vi "UHR-Fleezers Control (host) - 12.4.vi"() -> ()   [LabVIEW 2012] (continued)
        n2469 = Build Array (concatenate)(w3745, w3711) -> (w3744:dbl[])
        n2470 = Select(t=w3713, s=w3710, f=w3772) -> (s? t:f=w3757:dbl[])
        n2471 = feedback-in #11(w3757) -> ()
        n2472 = Select(t=w3711, s=w3710, f=w3744) -> (s? t:f=w3729:dbl[])
        n2473 = feedback-in #12(w3729) -> ()
        n2474 = feedback #13(w3715) -> (w3866:dbl[])
        n2475 = Build Array (concatenate)(w3866, w3715) -> (w3848:dbl[])
        n2476 = Select(t=w3715, s=w3710, f=w3848) -> (s? t:f=w3852:dbl[])
        n2477 = feedback-in #13(w3852) -> ()
        n2478 = feedback #14(w3797) -> (w3854:dbl[])
        n2479 = Build Array (concatenate)(w3854, w3797) -> (w3845:dbl[])
        n2480 = feedback #15(w3804) -> (w3864:dbl[])
        n2481 = Build Array (concatenate)(w3864, w3804) -> (w3863:dbl[])
        n2482 = feedback #16(w3799) -> (w3856:dbl[])
        n2483 = Build Array (concatenate)(w3856, w3799) -> (w3857:dbl[])
        n2484 = Select(t=w3797, s=w3710, f=w3845) -> (s? t:f=w3801:dbl[])
        n2485 = feedback-in #14(w3801) -> ()
        n2486 = Select(t=w3804, s=w3710, f=w3863) -> (s? t:f=w3803:dbl[])
        n2487 = feedback-in #15(w3803) -> ()
        n2488 = Select(t=w3799, s=w3710, f=w3857) -> (s? t:f=w3802:dbl[])
        n2489 = feedback-in #16(w3802) -> ()
        n2490 = call "integrate 1D array interval - double.vi"("Ave N"=w3709, "Array In"=w3757) -> ("Array Out"=w3768:dbl[])  [unwired: 1 out]
        n2491 = call "integrate 1D array interval - double.vi"("Ave N"=w3709, "Array In"=w3729) -> ("Array Out"=w3740:dbl[])  [unwired: 1 out]
        n2492 = call "integrate 1D array interval - double.vi"("Ave N"=w3709, "Array In"=w3852) -> ("Array Out"=w3851:dbl[])  [unwired: 1 out]
        n2493 = Array Size(array=w3768) -> (size(s)=w3769:i32)
        n2494 = Array Size(array=w3740) -> (size(s)=w3741:i32)
        n2495 = Array Size(array=w3851) -> (size(s)=w3853:i32)
        n2496 = Multiply(x=w3707, y=w3708) -> (x*y=w3771:u64)
        n2497 = Multiply(x=w3707, y=w3708) -> (x*y=w3743:u64)
        n2498 = Multiply(x=w3707, y=w3708) -> (x*y=w3861:u64)
        n2499 = Subtract(x=w3771, y=w3769) -> (x-y=w3762:u64)
        n2500 = call-poly <vilib>:"Mean.vi"("X"=w3768) -> ("mean"=w3759:dbl)  [unwired: 1 out]
        n2501 = Subtract(x=w3743, y=w3741) -> (x-y=w3734:u64)
        n2502 = call-poly <vilib>:"Mean.vi"("X"=w3740) -> ("mean"=w3731:dbl)  [unwired: 1 out]
        n2503 = Subtract(x=w3861, y=w3853) -> (x-y=w3795:u64)
        n2504 = call-poly <vilib>:"Mean.vi"("X"=w3851) -> ("mean"=w3792:dbl)  [unwired: 1 out]
        n2505 = call-poly <vilib>:"Mean.vi"("X"=w3801) -> ("mean"=w3785:dbl)  [unwired: 1 out]
        n2506 = call-poly <vilib>:"Mean.vi"("X"=w3803) -> ("mean"=w3790:dbl)  [unwired: 1 out]
        n2507 = call-poly <vilib>:"Mean.vi"("X"=w3802) -> ("mean"=w3788:dbl)  [unwired: 1 out]
        n2508 = Initialize Array(1.0 ("element"), w3762) -> (w3758:dbl[])
        n2509 = Initialize Array(1.0 ("element"), w3734) -> (w3730:dbl[])
        n2510 = Initialize Array(1.0 ("element"), w3795) -> (w3786:dbl[])
        n2511 = Multiply(x=w3758, y=w3759) -> (x*y=w3760:dbl[])
        n2512 = Multiply(x=w3730, y=w3731) -> (x*y=w3732:dbl[])
        n2513 = Multiply(x=w3786, y=w3792) -> (x*y=w3793:dbl[])
        n2514 = Multiply(x=w3786, y=w3788) -> (x*y=w3789:dbl[])
        n2515 = Multiply(x=w3786, y=w3790) -> (x*y=w3791:dbl[])
        n2516 = Multiply(x=w3786, y=w3785) -> (x*y=w3787:dbl[])
        n2517 = Build Array (concatenate)(w3768, w3760) -> (w3770:dbl[])
        n2518 = Build Array (concatenate)(w3740, w3732) -> (w3742:dbl[])
        n2519 = Build Array (concatenate)(w3851, w3793) -> (w3860:dbl[])
        n2520 = Build Array (concatenate)(w3801, w3787) -> (w3855:dbl[])
        n2521 = Build Array (concatenate)(w3803, w3791) -> (w3859:dbl[])
        n2522 = Build Array (concatenate)(w3802, w3789) -> (w3858:dbl[])
        n2523 = Reshape Array(w3770, w3707, w3708) -> (w3766:dbl[][])
        n2524 = Reshape Array(w3742, w3707, w3708) -> (w3738:dbl[][])
        n2525 = Reshape Array(w3860, w3707, w3708) -> (w3838:dbl[][])
        n2526 = Reshape Array(w3855, w3707, w3708) -> (w3821:dbl[][])
        n2527 = Reshape Array(w3859, w3707, w3708) -> (w3813:dbl[][])
        n2528 = Reshape Array(w3858, w3707, w3708) -> (w3828:dbl[][])
        n2529 = Array Subset(array=w3766, index (col)=0 ("index"), length (col)=w3706) -> (w3765:dbl[][])  [unwired: 2 in]
        n2530 = Array Subset(array=w3766, index (col)=w3706) -> (w3763:dbl[][])  [unwired: 3 in]
        n2531 = Array Subset(array=w3738, index (col)=0 ("index"), length (col)=w3706) -> (w3737:dbl[][])  [unwired: 2 in]
        n2532 = Array Subset(array=w3738, index (col)=w3706) -> (w3735:dbl[][])  [unwired: 3 in]
        n2533 = Array Subset(array=w3828, index (col)=0 ("index"), length (col)=w3706) -> (w3833:dbl[][])  [unwired: 2 in]
        n2534 = Array Subset(array=w3828, index (col)=w3706) -> (w3831:dbl[][])  [unwired: 3 in]
        n2535 = Array Subset(array=w3838, index (col)=0 ("index"), length (col)=w3706) -> (w3837:dbl[][])  [unwired: 2 in]
        n2536 = Array Subset(array=w3838, index (col)=w3706) -> (w3835:dbl[][])  [unwired: 3 in]
        n2537 = Array Subset(array=w3813, index (col)=0 ("index"), length (col)=w3706) -> (w3819:dbl[][])  [unwired: 2 in]
        n2538 = Array Subset(array=w3813, index (col)=w3706) -> (w3817:dbl[][])  [unwired: 3 in]
        n2539 = Array Subset(array=w3821, index (col)=0 ("index"), length (col)=w3706) -> (w3826:dbl[][])  [unwired: 2 in]
        n2540 = Array Subset(array=w3821, index (col)=w3706) -> (w3824:dbl[][])  [unwired: 3 in]
        n2541 = for {
          tunnel: w3765 -> [w3870] mode=indexing
          tunnel: [w3869] -> w3764 mode=indexing
          workers-P: _ -> [_]
          n2542 = Reverse 1D Array(array=w3870) -> (reversed array=w3869:dbl[])
        }
        n2543 = for {
          tunnel: w3737 -> [w3868] mode=indexing
          tunnel: [w3867] -> w3736 mode=indexing
          workers-P: _ -> [_]
          n2544 = Reverse 1D Array(array=w3868) -> (reversed array=w3867:dbl[])
        }
        n2545 = for {
          tunnel: w3833 -> [w3876] mode=indexing
          tunnel: [w3875] -> w3832 mode=indexing
          workers-P: _ -> [_]
          n2546 = Reverse 1D Array(array=w3876) -> (reversed array=w3875:dbl[])
        }
        n2547 = for {
          tunnel: w3837 -> [w3878] mode=indexing
          tunnel: [w3877] -> w3836 mode=indexing
          workers-P: _ -> [_]
          n2548 = Reverse 1D Array(array=w3878) -> (reversed array=w3877:dbl[])
        }
        n2549 = for {
          tunnel: w3819 -> [w3872] mode=indexing
          tunnel: [w3871] -> w3818 mode=indexing
          workers-P: _ -> [_]
          n2550 = Reverse 1D Array(array=w3872) -> (reversed array=w3871:dbl[])
        }
        n2551 = for {
          tunnel: w3826 -> [w3874] mode=indexing
          tunnel: [w3873] -> w3825 mode=indexing
          workers-P: _ -> [_]
          n2552 = Reverse 1D Array(array=w3874) -> (reversed array=w3873:dbl[])
        }
        n2553 = Index Array(array=w3838, index (row)=0) -> (element=→"Waveform Graph":dbl[])  [unwired: 1 in]
        n2554 = Add(x=w3764, y=w3763) -> (x+y=w3750:dbl[][])
        n2555 = Add(x=w3736, y=w3735) -> (x+y=w3722:dbl[][])
        n2556 = Add(x=w3832, y=w3831) -> (x+y=w3830:dbl[][])
        n2557 = Add(x=w3836, y=w3835) -> (x+y=w3810:dbl[][])
        n2558 = Add(x=w3818, y=w3817) -> (x+y=w3816:dbl[][])
        n2559 = Add(x=w3825, y=w3824) -> (x+y=w3823:dbl[][])
        n2560 = Divide(x=w3816, y=2) -> (x/y=w3814:dbl[][])
        n2561 = Divide(x=w3830, y=2) -> (x/y=w3775:dbl[][])
        n2562 = To Single Precision Float(number=w3810) -> (single precision float=w3809:sgl[][])
        n2563 = To Single Precision Float(number=w3750) -> (single precision float=w3754:sgl[][])
        n2564 = To Single Precision Float(number=w3722) -> (single precision float=w3726:sgl[][])
        n2565 = Divide(x=w3823, y=2) -> (x/y=w3777:dbl[][])
        n2566 = Transpose 2D Array(2D array=w3814) -> (transposed array=→"Data map":dbl[][])
        n2567 = To Single Precision Float(number=w3775) -> (single precision float=w3781:sgl[][])
        n2568 = To Single Precision Float(number=w3777) -> (single precision float=w3778:sgl[][])
        n2569 = call "IMAQ ArrayToImage"("Image Pixels (Float)"=w3809, "Image"=w3747) -> ("Image Out"=w3812:T2)  [unwired: 8 in, 1 out]
        n2570 = call "IMAQ ArrayToImage"("Image Pixels (Float)"=w3754, "Image"=w3746) -> ("Image Out"=w3756:T2)  [unwired: 8 in, 1 out]
        n2571 = call "IMAQ ArrayToImage"("Image Pixels (Float)"=w3726, "Image"=w3718) -> ("Image Out"=w3728:T2)  [unwired: 8 in, 1 out]
        n2572 = call "IMAQ ArrayToImage"("Image Pixels (Float)"=w3781, "Image"=w3719) -> ("Image Out"=w3783:T2)  [unwired: 8 in, 1 out]
        n2573 = call "IMAQ Symmetry"("Type of Symmetry"=w3811, "Image Src"=w3812) -> ("Image Dst Out"=w3807:T2)  [unwired: 3 in, 1 out]
        n2574 = call "IMAQ ArrayToImage"("Image Pixels (Float)"=w3778, "Image"=w3720) -> ("Image Out"=w3780:T2)  [unwired: 8 in, 1 out]
        n2575 = call "IMAQ Symmetry"("Type of Symmetry"=w3755, "Image Src"=w3756) -> ("Image Dst Out"=w3752:T2)  [unwired: 3 in, 1 out]
        n2576 = call "IMAQ Symmetry"("Type of Symmetry"=w3727, "Image Src"=w3728) -> ("Image Dst Out"=w3724:T2)  [unwired: 3 in, 1 out]
        n2577 = call "IMAQ Symmetry"("Type of Symmetry"=w3782, "Image Src"=w3783) -> ("Image Dst Out"=→"Detection Laser X":T2)  [unwired: 3 in, 1 out]
        n2578 = call "IMAQ Symmetry"("Type of Symmetry"=w3779, "Image Src"=w3780) -> ("Image Dst Out"=→"Detection Laser Y":T2)  [unwired: 3 in, 1 out]
        n2579 = call "IMAQ Set Simple Calibration"("Calibration Axis Info"=T34 {"Origin Pixel"={"X"=0.0, "Y"=0.0}, "Angle Relative to Horizontal (deg)"=0.0, "Axis Reference"=0}, "Grid Descriptor"=T35 {"X Step"=0.3, "Y Step"=0.3, "Unit"=enum."Undefined"}, "Image"=w3807) -> ("Calibrated Image"=→"APD 1":T2)  [unwired: 7 in, 1 out]
        n2580 = call "IMAQ Set Simple Calibration"("Calibration Axis Info"=T34 {"Origin Pixel"={"X"=0.0, "Y"=0.0}, "Angle Relative to Horizontal (deg)"=0.0, "Axis Reference"=0}, "Grid Descriptor"=T35 {"X Step"=0.3, "Y Step"=0.3, "Unit"=enum."Undefined"}, "Image"=w3752) -> ("Calibrated Image"=→"APD 2":T2)  [unwired: 7 in, 1 out]
        n2581 = call "IMAQ Set Simple Calibration"("Calibration Axis Info"=T34 {"Origin Pixel"={"X"=0.0, "Y"=0.0}, "Angle Relative to Horizontal (deg)"=0.0, "Axis Reference"=0}, "Grid Descriptor"=T35 {"X Step"=0.3, "Y Step"=0.3, "Unit"=enum."Undefined"}, "Image"=w3724) -> ("Calibrated Image"=→"APD 3":T2)  [unwired: 7 in, 1 out]
      }
    }
    n2582 = case "For computing FFTs for display" shown="True" "Compute FFT" {
      tunnel: w3218 -> [_ w4350]
      frame False {
      }
      frame True {
        n2583 = Build Array("FFT 1 Choice 1", "FFT 1 Choice 2", "FFT 2 Choice 1", "FFT 2 Choice 2") -> (w4343:u16[])
        n2584 = Array Size(array=w4350) -> (size(s)=w4349:i32)
        n2585 = feedback-in #17(w4343) -> ()
        n2586 = feedback #17(u16[] [100, 100, 100, 100]) -> (w4344:u16[])
        n2587 = feedback-in #18("# Spectra to Ave.") -> ()
        n2588 = feedback #18("# Spectra to Ave.") -> (w4341:dbl)
        n2589 = Not Equal?(x="# Spectra to Ave.", y=w4341) -> (x != y?=w4340:bool)
        n2590 = Not Equal?(x=w4343, y=w4344) -> (x != y?=w4342:bool)
        n2591 = feedback #19(1.0) -> (w4327:dbl)
        n2592 = Compound Arithmetic op=OR("Reset FFT", w4342, w4340) -> (w4325:bool)
        n2593 = Select(t=1.0, s=w4325, f=w4327) -> (s? t:f=w4329:dbl)
        n2594 = Greater?(x=w4329, y="# Spectra to Ave.") -> (0:w4348:bool)
        n2595 = Increment(x=w4329) -> (x+1=w4328:dbl)
        n2596 = feedback-in #19(w4328) -> ()
        n2597 = local read "DMA Update Period (s)"() -> (w4323:dbl)
        n2598 = Multiply(x="# Spectra to Ave.", y=w4323) -> (x*y=→"Ave. Time (s)":dbl)
        n2599 = Build Array(cluster{"f0":dbl, "df":dbl, "magnitude":dbl[]} {"f0"=0.0, "df"=0.0, "magnitude"=[]} ("PSD")) -> (w4332:cluster{"f0":dbl, "df":dbl, "magnitude":dbl[]}[])
        n2600 = Build Array(w4332, w4332, w4332, w4332) -> (w4334:T44)
        n2601 = feedback #20(w4334) -> (w4339:T44)
        n2602 = for {
          N: 4 -> [_]
          tunnel: w4343 -> [w4372] mode=indexing
          tunnel: w4350 -> [w4373]
          tunnel: w4349 -> [w4375]
          tunnel: w4325 -> [w4368]
          tunnel: w4348 -> [w4367]
          tunnel: "# Spectra to Ave." -> [w4366]
          tunnel: [w4365] -> w4338 mode=indexing
          tunnel: w4339 -> [w4370] mode=indexing
          tunnel: [w4369] -> w4326 mode=indexing
          tunnel: w4329 -> [w4364]
          n2603 = Less?(x=w4372, y=w4375) -> (x < y?=w4374:bool)
          n2604 = Index Array(array=w4373, index=w4372) -> (element=w4371:waveform(dbl))
          n2605 = case shown="True" w4374 {
            tunnel: w4371 -> [_ w4392]
            tunnel: w4370 -> [w4377 w4390]
            tunnel: [w4377 w4378] -> w4369
            tunnel: w4368 -> [_ w4389]
            tunnel: w4367 -> [_ w4382]
            tunnel: w4366 -> [_ w4381]
            tunnel: [cluster{"f0":dbl, "df":dbl, "magnitude":dbl[]} {"f0"=0.0, "df"=0.0, "magnitude"=[]} ("PSD") w4383] -> w4365
            tunnel: w4364 -> [_ w4380]
            frame False {
            }
            frame True {
              n2606 = call <vilib>:"Std Deviation and Variance.vi"("X"=w4392) -> ("mean"=w4393:dbl)  [unwired: 1 in, 2 out]
              n2607 = Subtract(x=w4392, y=w4393) -> (x-y=w4391:waveform(dbl))
              n2608 = xnode "Spectral Measurements"("Signals"=w4391) -> ("PSD"=w4385:cluster{"f0":dbl, "df":dbl, "magnitude":dbl[]})  [unwired: 1 in, 1 out]
              n2609 = case shown="False" w4389 {
                tunnel: w4390 -> [w4402 _]
                tunnel: [w4398 w4407] -> w4378
                tunnel: w4385 -> [w4401 w4408]
                tunnel: w4382 -> [w4400 _]
                frame False {
                  n2610 = Build Array (concatenate)(w4402, w4401) -> (w4399:cluster{"f0":dbl, "df":dbl, "magnitude":dbl[]}[])
                  n2611 = case shown="True" w4400 {
                    tunnel: w4399 -> [w4403 w4406]
                    tunnel: [w4403 w4404] -> w4398
                    frame False {
                    }
                    frame True {
                      n2612 = Delete From Array(array=w4406, index=0) -> (array with subset deleted=w4404:cluster{"f0":dbl, "df":dbl, "magnitude":dbl[]}[])  [unwired: 1 in, 1 out]
                    }
                  }
                }
                frame True {
                  n2613 = Build Array(w4408) -> (w4407:cluster{"f0":dbl, "df":dbl, "magnitude":dbl[]}[])
                }
              }
              n2614 = for {
                tunnel: w4378 -> [w4397] mode=indexing
                tunnel: [w4396] -> w4388 mode=indexing
                workers-P: _ -> [_]
                n2615 = Unbundle By Name(w4397) -> ("magnitude"=w4396:dbl[])
              }
              n2616 = Transpose 2D Array(2D array=w4388) -> (transposed array=w4387:dbl[][])
              n2617 = for {
                tunnel: w4387 -> [w4395] mode=indexing
                tunnel: [w4394] -> w4386 mode=indexing
                workers-P: _ -> [_]
                n2618 = Add Array Elements(numeric array=w4395) -> (sum=w4394:dbl)
              }
              n2619 = Select(t=w4381, s=w4382, f=w4380) -> (s? t:f=w4379:dbl)
              n2620 = Divide(x=w4386, y=w4379) -> (x/y=w4384:dbl[])
              n2621 = Bundle By Name(cluster=w4385, "magnitude"=w4384) -> (w4383:cluster{"f0":dbl, "df":dbl, "magnitude":dbl[]})
            }
          }
        }
        n2622 = case shown="True" w4325 {
          tunnel: w4326 -> [w4357 w4363]
          tunnel: [w4357 w4358] -> w4324
          frame False {
          }
          frame True {
            n2623 = Array Subset(array=w4363, index (row)=0 ("index"), length (row)=4 ("length"), index (col)=0 ("index"), length (col)=1 ("length")) -> (w4358:T44)
          }
        }
        n2624 = feedback-in #20(w4324) -> ()
        n2625 = Split 1D Array(array=w4338, index=2) -> (first subarray=→"FFT 1":cluster{"f0":dbl, "df":dbl, "magnitude":dbl[]}[], second subarray=→"FFT 2":cluster{"f0":dbl, "df":dbl, "magnitude":dbl[]}[])
      }
    }
    n2626 = Index Array(array=w3216, index=4) -> (element=w3272:waveform(dbl))
    n2627 = Index Array(array=w3216, index=7) -> (element=w3269:waveform(dbl))
    n2628 = Divide(x="T1 offset_x (mV)", y=1000.0) -> (x/y=w3273:dbl)
    n2629 = feedback-in #21("Calibration") -> ()
    n2630 = feedback #21(u16 1 ("Calibration")) -> (w3291:u16)
    n2631 = Divide(x="T2 offset_x (mV)", y=1000.0) -> (x/y=w3271:dbl)
    n2632 = case shown="2" "Calibration" {
      tunnel: "T1 alpha_x (nm/V)" -> [_ w3671 w3692]
      tunnel: "T1 kappa_x (pN/nm)" -> [_ _ w3682]
      tunnel: "T2 alpha_x (nm/V)" -> [_ w3670 w3690]
      tunnel: "T2 kappa_x (pN/nm)" -> [_ _ w3683]
      tunnel: w3272 -> [w3653 w3668 w3688]
      tunnel: w3269 -> [w3652 w3666 w3686]
      tunnel: [w3653 w3665 w3685] -> w3300
      tunnel: [w3652 w3664 w3684] -> w3299
      tunnel: ["T1 X (V)" ("Label.Text") "T1 X (nm)" ("Label.Text") "T1 X (pN)" ("Label.Text")] -> w3288
      tunnel: ["T2 X (V)" ("Label.Text") "T2 X (nm)" ("Label.Text") "T2 X (pN)" ("Label.Text")] -> w3287
      tunnel: ["Position (V)" ("Label.Text") "Position (nm)" ("Label.Text") "Force (pN)" ("Label.Text")] -> w3289
      tunnel: w3271 -> [_ w3656 w3675]
      tunnel: w3273 -> [_ w3659 w3677]
      tunnel: ["Mean (V)" ("Label.Text") "Mean (nm)" ("Label.Text") "Mean (pN)" ("Label.Text")] -> w3284
      tunnel: ["Difference (V)" ("Label.Text") "Difference (nm)" ("Label.Text") "Difference (pN)" ("Label.Text")] -> w3224
      frame 0, Default {
      }
      frame 1 {
        n2633 = Unbundle By Name(w3668) -> ("Y"=w3672:dbl[])
        n2634 = Unbundle By Name(w3666) -> ("Y"=w3657:dbl[])
        n2635 = Subtract(x=w3672, y=w3659) -> (x-y=w3660:dbl[])
        n2636 = Subtract(x=w3657, y=w3656) -> (x-y=w3658:dbl[])
        n2637 = Multiply(x=w3658, y=w3670) -> (x*y=w3667:dbl[])
        n2638 = Multiply(x=w3671, y=w3660) -> (x*y=w3669:dbl[])
        n2639 = Bundle By Name(cluster=w3666, "Y"=w3667) -> (w3664:waveform(dbl))
        n2640 = Bundle By Name(cluster=w3668, "Y"=w3669) -> (w3665:waveform(dbl))
      }
      frame 2 {
        n2641 = Unbundle By Name(w3688) -> ("Y"=w3693:dbl[])
        n2642 = Unbundle By Name(w3686) -> ("Y"=w3691:dbl[])
        n2643 = Subtract(x=w3691, y=w3675) -> (x-y=w3676:dbl[])
        n2644 = Subtract(x=w3693, y=w3677) -> (x-y=w3678:dbl[])
        n2645 = Compound Arithmetic op=MULTIPLY(w3676, w3690, w3683) -> (w3687:dbl[])
        n2646 = Compound Arithmetic op=MULTIPLY(w3682, w3692, w3678) -> (w3689:dbl[])
        n2647 = Bundle By Name(cluster=w3686, "Y"=w3687) -> (w3684:waveform(dbl))
        n2648 = Bundle By Name(cluster=w3688, "Y"=w3689) -> (w3685:waveform(dbl))
      }
    }
    n2649 = case shown="True" "Read Lateness and Rel Phase" {
      tunnel: w3090 -> [w3602 w3641]
      tunnel: w3089 -> [w3603 w3640]
      tunnel: [w3602 w3607] -> w3266
      tunnel: [w3603 w3606] -> w3265
      frame False {
      }
      frame True {
        n2650 = xnode "Read/Write Control"("FPGA VI Reference In"=w3641, "error in"=w3640) -> ("FPGA VI Reference Out"=w3609:T19, "error out"=w3608:errorcluster, "GI Relative phase"=→"GI relative phase":i16, "Relative phase"=→"Relative phase (AI1)":i16, "AI Late Counter"=→"Late Counter (AI1)":u8, "GI Late Counter"=→"GI Late Counter":u8, "MCL Late Counter"=→"MCL Late Counter":u8, "MCL Relative Phase"=→"Relative Phase (MCL)":i16, "APD Acq Relative Phase"=→"APD Acq Relative Phase":i16, "APD 1 Gate Relative Phase"=→"APD 1 Gate Relative Phase":i16, "APD 2 Gate Relative Phase"=→"APD 2 Gate Relative Phase":i16, "APD Acq Late Counter"=→"APD Acq Late Counter":u8, "APD 1 Gate Late Counter"=→"APD 1 Gate Late Counter":u8, "APD 2 Gate Late Counter"=→"APD 2 Gate Late Counter":u8, "Green FB Relative Phase"=→"Relative phase (Green FB)":i16, "GI Relative phase 2"=→"GI relative phase 2":i16, "GI Late Counter 2"=→"GI Late Counter 2":u8, "Trap Pos FIFO Timeout"=→"Trap Pos FIFO Timeout":u16, "Trap AI FIFO Timeout"=→"Trap AI FIFO Timeout":u16, "RI Late Counter"=→"RI Late Counter":u8, "RI Late Counter 2"=→"RI Late Counter 2":u8, "RI Relative phase"=→"RI relative phase":i16, "RI Relative phase 2"=→"RI relative phase 2":i16, "Red FB Relative Phase"=→"Relative phase (RI FB)":i16, "Red Late Counter"=→"Red AI Late Counter":u8, "Green Late Counter"=→"Green AI Late Counter":u8, "BI Late Counter (AO)"=→"Late Counter (BI AO)":u8, "Blue Late Counter (D)"=→"Late Counter (BI DO)":u8, "Blue Int Late Counter"=→"Late Counter (BI AI)":u8, "Blue Int Relative Phase"=→"Relative phase (BI AI)":i16, "BI Relative phase (AO)"=→"Relative phase (BI AO)":i16, "BI Relative phase (D)"=→"Relative phase (BI DO)":i16)
        n2651 = xnode "Read/Write Control"("FPGA VI Reference In"=w3609, "error in"=w3608) -> ("FPGA VI Reference Out"=w3607:T19, "error out"=w3606:errorcluster, "APD 3 Gate Late Counter"=→"APD 3 Gate Late Counter":u8, "APD 3 Gate Relative Phase"=→"APD 3 Gate Relative Phase":i16)
      }
    }
    n2652 = Not Equal?(x=w3291, y="Calibration") -> (x != y?=w3250:bool)
    n2653 = case shown="True" w3250 {
      tunnel: w3289 -> [_ w3646]
      tunnel: w3288 -> [_ w3645]
      tunnel: w3287 -> [_ w3644]
      tunnel: w3284 -> [_ w3643]
      tunnel: w3224 -> [_ w3642]
      frame False {
      }
      frame True {
        n2654 = property on="Force" class="WFChart (strict)"("YScale.NameLbl.Text"=w3646) -> ()  [unwired: 2 in, 2 out]
        n2655 = property on="T2 X" class="DigNum (strict)"("Caption.Text"=w3644) -> ()  [unwired: 2 in, 2 out]
        n2656 = property on="T1 X" class="DigNum (strict)"("Caption.Text"=w3645) -> ()  [unwired: 2 in, 2 out]
        n2657 = property on="Mean" class="DigNum (strict)"("Caption.Text"=w3643) -> ()  [unwired: 2 in, 2 out]
        n2658 = property on="Difference" class="DigNum (strict)"("Caption.Text"=w3642) -> ()  [unwired: 2 in, 2 out]
      }
    }
    n2659 = Unbundle By Name(w3272) -> ("Y"=w3275:dbl[])
    n2660 = Unbundle By Name(w3269) -> ("Y"=w3278:dbl[])
    n2661 = Subtract(x=w3275, y=w3273) -> (x-y=w3276:dbl[])
    n2662 = Subtract(x=w3278, y=w3271) -> (x-y=w3277:dbl[])
    n2663 = Multiply(x=w3277, y="T2 alpha_x (nm/V)") -> (x*y=w3072:dbl[])
    n2664 = Multiply(x="T1 alpha_x (nm/V)", y=w3276) -> (x*y=w3073:dbl[])
    n2665 = Not(x="Trap Trig. Fl.") -> (.not. x?=w3109:bool)
    n2666 = Multiply(x=w3299, y=-1.0) -> (x*y=w3280:waveform(dbl))
    n2667 = Subtract(x=w3073, y=w3072) -> (x-y=w3268:dbl[])
    n2668 = Unbundle By Name(w3299) -> ("Y"=w3240:dbl[])
    n2669 = Unbundle By Name(w3300) -> ("Y"=w3074:dbl[])
    n2670 = Negate(x=w3268) -> (-x=w3070:dbl[])
    n2671 = Build Array(w3300, w3280) -> (→"Force":waveform(dbl)[])
    n2672 = Subtract(x=w3070, y="Offset (nm)") -> (x-y=w3238:dbl[])
    n2673 = call-poly <vilib>:"Mean.vi"("X"=w3240) -> ("mean"=w3076:dbl)  [unwired: 1 out]
    "T2 X" <- w3076
    n2674 = Negate(x=w3240) -> (-x=w3241:dbl[])
    n2675 = call-poly <vilib>:"Mean.vi"("X"=w3074) -> ("mean"=w3077:dbl)  [unwired: 1 out]
    "T1 X" <- w3077
    n2676 = Negate(x=w3076) -> (-x=w3075:dbl)
    n2677 = Bundle By Name(cluster=w3272, "Y"=w3238) -> (w3215:waveform(dbl))
    "Bead Separation" <- w3215
    n2678 = Add(x=w3074, y=w3241) -> (x+y=w3242:dbl[])
    n2679 = Add(x=w3077, y=w3075) -> (x+y=w3286:dbl)
    n2680 = Subtract(x=w3077, y=w3075) -> (x-y=→"Difference":dbl)
    n2681 = Divide(x=w3242, y=2.0) -> (x/y=→"Vec Mean of T1 T2":dbl[])
    n2682 = Divide(x=w3286, y=2.0) -> (x/y=w3244:dbl)
    "Mean" <- w3244
    n2683 = feedback-in #22("Trap Trig. Fl.") -> ()
    n2684 = feedback #22("Trap Trig. Fl.") -> (w3107:bool)
    n2685 = And(x=w3109, y=w3107) -> (x .and. y?=w3108:bool)
    n2686 = case "If have just turned off triggering" shown="True" w3108 {
      tunnel: w3090 -> [_ w3437]
      tunnel: w3089 -> [_ w3436]
      frame False {
      }
      frame True {
        w3435 = FALSE ("FPGA Trap Trig")
        n2687 = xnode "Read/Write Control"("FPGA VI Reference In"=w3437, "error in"=w3436, "FPGA Trap Trig"=w3435) -> ("FPGA VI Reference Out"=w3434:T19, "error out"=w3433:errorcluster)
        n2688 = xnode "Read/Write Control"("FPGA VI Reference In"=w3434, "error in"=w3433, "TTrig?"=w3435) -> ()  [unwired: 2 out]
        n2689 = local write "Initializing"(FALSE ("Initializing")) -> ()
        n2690 = local write "Triggered"(FALSE ("Triggered")) -> ()
        n2691 = local write "Waiting"(FALSE ("Waiting")) -> ()
      }
    }
    n2692 = Not(x=w3107) -> (.not. x?=w3120:bool)
    n2693 = And(x="Trap Trig. Fl.", y=w3120) -> (x .and. y?=w3117:bool)
    n2694 = local read "Tether"() -> (w3245:bool)
    n2695 = Or(x=w3117, y="Reinitialize") -> (x .or. y?=w3103:bool)
    n2696 = feedback #23(w3113) -> (w3118:string)
    n2697 = Select(t=w3113, s=w3117, f=w3118) -> (s? t:f=w3112:string)
    n2698 = Select(t=w3113, s="Reinitialize", f=w3112) -> (s? t:f=w3111:string)
    n2699 = feedback #24(0) -> (w3115:i32)
    n2700 = feedback #25(w3238) -> (w3237:dbl[])
    n2701 = Build Array (concatenate)(w3238, w3237) -> (w3071:dbl[])
    n2702 = case "For determining if there is a tether still" shown="True" w3245 {
      tunnel: w3244 -> [_ w3561]
      frame False {
      }
      frame True {
        n2703 = Greater?(x="Lost Tether Alarm Threshold (pN)", y=w3561) -> (0:w3559:bool)
        n2704 = case shown="True" w3559 {
          frame False {
          }
          frame True {
            w3562 = FALSE ("Value (Signaling)")
            n2705 = flat-sequence {
              frame #0 {
                # "stop only if saving"
                n2706 = local read "Saving..."() -> (w3574:bool)
                n2707 = And(x=w3574, y="TA Cancel Save?") -> (x .and. y?=w3573:bool)
                n2708 = local write "Stop Saving"(w3573) -> ()
              }
              frame #1 {
                n2709 = case shown="True" "TA Green Off?" {
                  frame False {
                  }
                  frame True {
                    w3577 = FALSE ("Fl. Triggered...")
                    n2710 = local write "Fl. Triggered..."(w3577) -> ()
                    n2711 = property on="Green Laser ON" class="Bool (strict)"("Val(Sgnl)"=w3577) -> ()  [unwired: 2 in, 2 out]
                  }
                }
              }
            }
            n2712 = local read "Time tether formed"() -> (w3568:timestamp)
            n2713 = Get Date/Time In Seconds() -> (seconds since 1Jan1904=w3569:timestamp)
            n2714 = Subtract(x=w3569, y=w3568) -> (x-y=w3567:dbl)
            n2715 = Number To Decimal String(number=w3567) -> (decimal integer string=w3564:string)  [unwired: 1 out]
            n2716 = local read "Messages"() -> (w3571:string)
            n2717 = call <vilib>:"Beep.vi"() -> ()  [unwired: 3 in, 9 out]
            n2718 = Concatenate Strings("Lost tether (" ("Message to add"), w3564, " s)." ("string")) -> (w3566:string)
            n2719 = local write "Tether"(FALSE ("Tether")) -> ()
            n2720 = call "Update messages.vi"("Message to add"=w3566, "Old message string"=w3571) -> ("New message string"=w3570:string)
            n2721 = local write "Messages"(w3570) -> ()
            n2722 = property on="Fl. Triggered..." class="Bool (strict)"("Val(Sgnl)"=w3562) -> ()  [unwired: 2 in, 2 out]
            n2723 = local write "Dip for Protein"(w3562) -> ()
            n2724 = property on="Trap Pos. FB ON" class="Bool (strict)"("Val(Sgnl)"=w3562) -> ()  [unwired: 2 in, 2 out]
            n2725 = property on="Trap Trig. Fl." class="Bool (strict)"("Val(Sgnl)"=w3562) -> ()  [unwired: 2 in, 2 out]
          }
        }
      }
    }
    n2726 = case "For triggering actions based on the trap position (e.g., turning the excitation laser on if trap under feedback moves so far)" shown="True" "Trap Trig. Fl." {
      tunnel: w3098 -> [_ w3450]
      tunnel: w3111 -> [_ w3449]
      tunnel: ["" ("t") w3448] -> w3119
      tunnel: w3103 -> [_ w3447]
      tunnel: [0 ("t") w3446] -> w3116
      tunnel: w3115 -> [_ w3445]
      tunnel: w3090 -> [_ w3444]
      tunnel: w3089 -> [_ w3443]
      frame False {
      }
      frame True {
        n2727 = case shown="\"Wait for trigger\"" w3449 {
          tunnel: w3450 -> [w3467 _ _ w3515]
          tunnel: [w3464 w3496 "" ("t") w3518] -> w3448
          tunnel: w3447 -> [_ _ _ w3506]
          tunnel: [w3463 w3493 0 ("t") w3507] -> w3446
          tunnel: w3445 -> [_ w3495 _ w3513]
          tunnel: w3444 -> [w3452 w3490 _ w3509]
          tunnel: w3443 -> [w3451 w3489 _ w3508]
          frame "Wait for trigger" {
            n2728 = local read "Trap Trig. (FPGA)"() -> (w3455:bool)
            n2729 = Subtract(x=w3467, y="Mean T1 Position\nto compare (nm)") -> (x-y=w3460:dbl[])
            n2730 = call <vilib>:"Std Deviation and Variance.vi"("X"=w3460) -> ("mean"=→"mean":dbl, "standard deviation"=→"standard\ndeviation":dbl)  [unwired: 1 in, 1 out]
            n2731 = Array Max & Min(array=w3460) -> (max value=→"max value":dbl, min value=→"min value":dbl)  [unwired: 2 out]
            n2732 = Greater?(x=w3460, y="Threshold (nm)") -> (0:w3470:bool[])
            n2733 = case shown="True" w3455 {
              tunnel: w3452 -> [_ w3476]
              tunnel: w3451 -> [_ w3475]
              tunnel: [FALSE ("TTrig?") w3474] -> w3458
              frame False {
              }
              frame True {
                n2734 = xnode "Read/Write Control"("FPGA VI Reference In"=w3476, "error in"=w3475) -> ("TTrig?"=w3474:bool)  [unwired: 2 out]
              }
            }
            n2735 = Or Array Elements(Boolean array=w3470) -> (logical OR=w3457:bool)
            n2736 = Select(t=w3458, s=w3455, f=w3457) -> (s? t:f=w3456:bool)
            n2737 = Not(x=w3455) -> (.not. x?=w3454:bool)
            n2738 = And(x=w3456, y=w3454) -> (x .and. y?=w3453:bool)
            n2739 = Select(t="Triggered", s=w3456, f="Wait for trigger") -> (s? t:f=w3464:string)
            n2740 = case shown="True" w3456 {
              tunnel: [0 0] -> w3463
              tunnel: w3452 -> [_ w3481]
              tunnel: w3451 -> [_ w3480]
              frame False {
                "Waiting" <- TRUE ("Waiting")
              }
              frame True {
                n2741 = xnode "Read/Write Control"("FPGA VI Reference In"=w3481, "error in"=w3480, "TTrig?"=FALSE) -> ()  [unwired: 2 out]
                n2742 = local read "Messages"() -> (w3484:string)
                n2743 = call <vilib>:"Beep.vi"() -> ()  [unwired: 12 in]
                n2744 = call "Update messages.vi"("Message to add"="Unwinding trigger.", "Old message string"=w3484) -> ("New message string"=w3485:string)
                n2745 = local write "Messages"(w3485) -> ()
                n2746 = local write "Waiting"(FALSE ("Waiting")) -> ()
                "Triggered" <- TRUE ("Triggered")
              }
            }
            n2747 = case "Only need to turn on laser if host triggered" shown="True" w3453 {
              frame False {
              }
              frame True {
                n2748 = property on="Green Laser ON" class="Bool (strict)"("Val(Sgnl)"=TRUE ("Value (Signaling)")) -> ()  [unwired: 2 in, 2 out]
              }
            }
          }
          frame "Triggered" {
            n2749 = local read "Trap Trig. (FPGA)"() -> (w3492:bool)
            n2750 = Increment(x=w3495) -> (x+1=w3493:i32)
            n2751 = Greater Or Equal?(x=w3493, y="Fl. ON time (n)") -> (x >= y?=w3491:bool)
            n2752 = Select(t="Wait for trigger", s=w3491, f="Triggered" ("t")) -> (s? t:f=w3496:string)
            n2753 = And(x=w3491, y=w3492) -> (x .and. y?=w3488:bool)
            n2754 = case shown="True" w3488 {
              tunnel: w3490 -> [_ w3500]
              tunnel: w3489 -> [_ w3499]
              frame False {
              }
              frame True {
                n2755 = xnode "Read/Write Control"("FPGA VI Reference In"=w3500, "error in"=w3499, "FPGA Trap Trig"=TRUE) -> ()  [unwired: 2 out]
              }
            }
            n2756 = case shown="True" w3491 {
              frame False {
              }
              frame True {
                w3502 = FALSE ("Value (Signaling)")
                n2757 = local write "Triggered"(w3502) -> ()
                n2758 = local write "Waiting"(TRUE ("Waiting")) -> ()
                n2759 = property on="Green Laser ON" class="Bool (strict)"("Val(Sgnl)"=w3502) -> ()  [unwired: 2 in, 2 out]
              }
            }
          }
          frame "Do nothing" {
          }
          frame "Initialize", Default {
            n2760 = Increment(x=w3513) -> (x+1=w3517:i32)
            n2761 = Select(t=1, s=w3506, f=w3517) -> (s? t:f=w3507:i32)
            n2762 = feedback #26(w3515) -> (w3521:dbl[])
            n2763 = Build Array (concatenate)(w3515, w3521) -> (w3514:dbl[])
            n2764 = Greater Or Equal?(x=w3507, y="Wait to get offset (n)") -> (x >= y?=w3510:bool)
            n2765 = Select(t=w3515, s=w3506, f=w3514) -> (s? t:f=w3516:dbl[])
            n2766 = feedback-in #26(w3516) -> ()
            n2767 = call-poly <vilib>:"Mean.vi"("X"=w3516) -> ("mean"=w3511:dbl)  [unwired: 1 out]
            n2768 = local write "Mean T1 Position\nto compare (nm)"(w3511) -> ()
            n2769 = case shown="True" w3506 {
              tunnel: w3509 -> [_ w3527]
              tunnel: w3508 -> [_ w3526]
              frame False {
              }
              frame True {
                w3523 = FALSE ("FPGA Trap Trig")
                n2770 = xnode "Read/Write Control"("FPGA VI Reference In"=w3527, "error in"=w3526, "FPGA Trap Trig"=w3523) -> ("FPGA VI Reference Out"=w3525:T19, "error out"=w3524:errorcluster)
                n2771 = xnode "Read/Write Control"("FPGA VI Reference In"=w3525, "error in"=w3524, "TTrig?"=w3523) -> ()  [unwired: 2 out]
              }
            }
            n2772 = Select(t="Wait for trigger", s=w3510, f="Initialize") -> (s? t:f=w3518:string)
            n2773 = case shown="True" w3510 {
              tunnel: w3511 -> [_ w3530]
              tunnel: w3509 -> [_ w3539]
              tunnel: w3508 -> [_ w3538]
              frame False {
                n2774 = local write "Waiting"(FALSE ("Waiting")) -> ()
                "Initializing" <- TRUE ("Initializing")
              }
              frame True {
                n2775 = local read "Threshold (nm)"() -> (w3542:dbl)
                n2776 = local read "AOM X Cal (nm/MHz)"() -> (w3541:dbl)
                n2777 = Add(x=w3530, y=w3542) -> (x+y=w3543:dbl)
                n2778 = Divide(x=w3543, y=w3541) -> (x/y=w3540:dbl)
                n2779 = call "IR AOM freq to word.vi"("Frequency In (MHz)"=w3540) -> ("Frequency Word Out (double)"=w3537:dbl)
                n2780 = local write "Initializing"(FALSE ("Initializing")) -> ()
                n2781 = local write "Waiting"(TRUE ("Waiting")) -> ()
                n2782 = To Quad Integer(1:w3537) -> (0:w3536:i64)
                n2783 = xnode "Read/Write Control"("FPGA VI Reference In"=w3539, "error in"=w3538, "FPGA TTrig Thresh"=w3536) -> ("FPGA VI Reference Out"=w3533:T19, "error out"=w3532:errorcluster)
                n2784 = xnode "Read/Write Control"("FPGA VI Reference In"=w3533, "error in"=w3532, "FPGA Trap Trig"=TRUE) -> ()  [unwired: 2 out]
              }
            }
          }
        }
      }
    }
    n2785 = feedback-in #23(w3119) -> ()
    n2786 = feedback-in #24(w3116) -> ()
    n2787 = Split 1D Array(array=w3071, index=w3133) -> (first subarray=w3234:dbl[])  [unwired: 1 out]
    n2788 = feedback-in #25(w3234) -> ()
    n2789 = call-poly <vilib>:"Mean.vi"("X"=w3234) -> ("mean"=w3233:dbl)  [unwired: 1 out]
    "Bead Mean (nm)" <- w3233
    n2790 = Subtract(x=w3234, y=w3233) -> (x-y=w3232:dbl[])
    n2791 = Square(x=w3232) -> (x^2=w3231:dbl[])
    n2792 = call-poly <vilib>:"Mean.vi"("X"=w3231) -> ("mean"=w3230:dbl)  [unwired: 1 out]
    n2793 = Square Root(x=w3230) -> (sqrt(x)=w3229:dbl)
    n2794 = Multiply(x=10.0, y=w3229) -> (x*y=→"RMS (Ang)":dbl)
    n2795 = xnode ("Read/Write Control")("FPGA VI Reference In"=w3266, "error in"=w3265) -> ("FPGA VI Reference Out"=w3101:T19, "error out"=w3100:errorcluster, "AI2 Y Sum Set 1"=w3364:i16, "AI2 Y Sum Set 2"=w3363:i16, "AI1 X Set 1"=w3165:fxp<+/-,16,1>, "AI1 X Set 2"=w3164:fxp<+/-,16,1>, "Trap Pos FB Int Signal"=→"Trap Pos FB Int Signal":fxp<+/-,24,9>, "Trap Pos FB Int-Norm Signal"=→"Trap Pos FB Int-Norm Signal":fxp<+/-,16,1>, "Trap Pos FB Action"=w3158:i64, "Scanning"=→"AOD Scanning":bool, "Scan I"=→"AOD Scan I":u64, "Scanning MCL"=w3366:bool, "Scan I (MCL)"=→"MCL Scan I":u64, "Green FB Sum"=w3303:i16, "Trap Pos FB Action"=w3088:i64, "TTrig Fin Thresh"=w3084:i64, "Red FB Intensity"=w3065:i16, "Blue Intensity"=w3060:i16)
    "MCL Scanning" <- w3366
    "Trap Pos FB Action" <- w3158
    n2796 = Divide(x=w3065, y=3276.7) -> (x/y=w3064:dbl)
    "Red laser intensity (V)" <- w3064
    n2797 = Divide(x=w3060, y=3276.7) -> (x/y=w3059:dbl)
    "Blue laser intensity (V)" <- w3059
    n2798 = Divide(x=w3303, y=3276.7) -> (x/y=w3063:dbl)
    "Green laser intensity (V)" <- w3063
    n2799 = local read "FB Trig Integrate"() -> (w3082:u32)
    n2800 = Divide(x=w3088, y=w3082) -> (x/y=w3081:dbl)
    "TTrig Sig (Int)" <- w3081
    n2801 = Bundle(w3063, w3064, w3059) -> (→"Fluorescence laser intensities plot":cluster{dbl, dbl, dbl})  [unwired: 1 in]
    n2802 = Divide(x=w3084, y=w3082) -> (x/y=w3079:dbl)
    "TTrig Fin Thresh (Int)" <- w3079
    n2803 = local read "AOM X Cal (nm/MHz)"() -> (w3087:dbl)
    n2804 = local read "AI2 (V)"() -> (w3365:cluster{"Set 1":dbl, "Set 2":dbl})
    n2805 = Bundle By Name(cluster=w3365, "Set 1"=w3364, "Set 2"=w3363) -> (w3361:cluster{"Set 1":dbl, "Set 2":dbl})
    n2806 = Divide(x=w3158, y=327.67) -> (x/y=→"Action (%)":dbl)
    n2807 = local read "Trap X (AI1)"() -> (w3178:T10)
    n2808 = call "IR AOM word double to freq.vi"("Frequency Word In (double)"=w3079) -> ("Frequency Out (MHz)"=w3078:dbl)
    n2809 = call "IR AOM word double to freq.vi"("Frequency Word In (double)"=w3081) -> ("Frequency Out (MHz)"=w3080:dbl)
    n2810 = Divide(x=w3361, y=3276.7) -> (x/y=w3360:cluster{"Set 1":dbl, "Set 2":dbl})
    n2811 = Multiply(x=w3080, y=w3087) -> (x*y=w3086:dbl)
    "TTrig Sig (nm)" <- w3086
    n2812 = Multiply(x=w3078, y=w3087) -> (x*y=w3085:dbl)
    "TTrig Fin Thresh (nm)" <- w3085
    n2813 = local write "AI2 (V)"(w3360) -> ()
    n2814 = Bundle(cluster=w3178, "Trap 1"=w3165, "Trap 2"=w3164) -> (→"Trap X (AI1)":T10)
    n2815 = Bundle(w3086, w3085) -> (→"TTrig":cluster{dbl, dbl})  [unwired: 1 in]
    n2816 = flat-sequence "To save data" {
      tunnel: [w4456] -> w3384
      tunnel: [w4457] -> w3383
      tunnel: w3334 -> [w4450]
      tunnel: w3106 -> [w4454]
      tunnel: ["Save Calibration"] -> w3357
      tunnel: w3354 -> [w4453]
      tunnel: [w4446] -> w3353
      tunnel: [w4443] -> w3352
      tunnel: [w4440] -> w3351
      tunnel: w3333 -> [w4442]
      tunnel: w3248 -> [w4436]
      tunnel: [w4436] -> w3247
      tunnel: ["Start Saving"] -> w3217
      tunnel: [w4430] -> w3146
      tunnel: [w4429] -> w3145
      tunnel: w3384 -> [w4693]
      tunnel: w3383 -> [w4692]
      tunnel: w3147 -> [w4691]
      tunnel: w3357 -> [w4690]
      tunnel: w3353 -> [w4688]
      tunnel: w3352 -> [w4687]
      tunnel: w3351 -> [w4686]
      tunnel: w3226 -> [w4685]
      tunnel: w3258 -> [w4684]
      tunnel: w3247 -> [w4683]
      tunnel: w3217 -> [w4682]
      tunnel: w3215 -> [w4681]
      tunnel: w3043 -> [w4680]
      tunnel: w3146 -> [w4679]
      tunnel: w3145 -> [w4678]
      tunnel: w3144 -> [w4677]
      tunnel: w3067 -> [w4676]
      frame #0 {
        n2817 = Or(x="Save N Sets", y="Start Saving") -> (x .or. y?=w4437:bool)
        n2818 = To Double Precision Float(number=w4453) -> (double precision float=w4447:dbl)
        n2819 = Build Array(w4437, "Save Calibration", w4450, w4442) -> (w4452:bool[])
        n2820 = Compound Arithmetic op=OR("Save Calibration", w4450, w4437, w4442) -> (w4455:bool)
        n2821 = Boolean Array To Number(Boolean array=w4452) -> (number=w4449:u32)
        n2822 = feedback #27(FALSE ("Save APD Data\nwith Trap Data")) -> (w4431:bool)
        n2823 = feedback #28(refnum<k0> refnum) -> (w4458:refnum<file>)
        n2824 = feedback #29(refnum<k0> refnum) -> (w4433:refnum<file>)
        n2825 = feedback #30(FALSE ("Save APD Data\nwith Trap Data")) -> (w4441:bool)
        n2826 = feedback #31(refnum<k0> refnum) -> (w4444:refnum<file>)
        n2827 = feedback #32(0) -> (w4460:i32)
        n2828 = feedback #33() -> (w4448:u32)  [unwired: 1 out]
        n2829 = case shown="True" w4455 {
          tunnel: [w4467 1] -> w4456
          tunnel: w4460 -> [w4469 _]
          tunnel: [w4468 w4487] -> w4457
          tunnel: w4458 -> [w4468 _]
          tunnel: w4454 -> [_ w4507]
          tunnel: w4447 -> [_ w4505]
          tunnel: w4449 -> [_ w4508]
          tunnel: [w4466 w4486] -> w4446
          tunnel: w4448 -> [w4466 _]
          tunnel: [w4465 w4484] -> w4443
          tunnel: w4444 -> [w4465 _]
          tunnel: [w4464 w4483] -> w4440
          tunnel: w4441 -> [w4464 _]
          tunnel: "Start Saving" -> [_ w4481]
          tunnel: w4436 -> [_ w4480]
          tunnel: [w4463 w4471] -> w4429
          tunnel: w4433 -> [w4463 _]
          tunnel: [w4462 w4470] -> w4430
          tunnel: w4431 -> [w4462 _]
          frame False {
            n2830 = Increment(x=w4469) -> (x+1=w4467:i32)
          }
          frame True {
            w4477 = FALSE ("Start Saving")
            w4482 = 9.0  # File Version
            w4490 = FALSE ("prepend array or string size? (T)")
            w4488 = T26."big-endian, network order" ("byte order (0:big-endian, network order)")
            n2831 = local read "BD 1 Frequency 1 (MHz)"() -> (w4504:dbl)
            n2832 = local read "BD 2 Frequency 1 (MHz)"() -> (w4503:dbl)
            n2833 = local read "BD 1 Frequency 2 (MHz)"() -> (w4502:dbl)
            n2834 = local read "BD 2 Frequency 2 (MHz)"() -> (w4501:dbl)
            n2835 = local read "BD 1 Frequency 3 (MHz)"() -> (w4500:dbl)
            n2836 = local read "BD 2 Frequency 3 (MHz)"() -> (w4499:dbl)
            n2837 = Array Size(array=w4480) -> (size(s)=w4479:i32)
            n2838 = To Double Precision Float(number=w4479) -> (double precision float=w4478:dbl)
            n2839 = local write "Save Calibration"(w4477) -> ()
            n2840 = local write "Start Saving"(w4477) -> ()
            n2841 = Build Array("Save APD Data\nwith Trap Data", "Save Trap Pos. Data") -> (w4474:bool[])
            n2842 = Boolean Array To Number(Boolean array=w4474) -> (number=w4473:u32)
            n2843 = Build Array(w4504, w4503, w4502, w4501, w4500, w4499) -> (w4498:dbl[])
            n2844 = case shown="1, Default" w4508 {
              tunnel: w4507 -> [w4580 w4600 w4616 w4654]
              tunnel: w4478 -> [w4585 w4607 w4636 w4673]
              tunnel: w4505 -> [w4584 w4606 w4635 w4672]
              tunnel: [w4581 w4602 w4627 w4664] -> w4496
              tunnel: [w4572 "Cal sets to save" w4617 w4655] -> w4486
              tunnel: w4498 -> [w4582 w4603 w4629 w4666]
              tunnel: "Save APD Data\nwith Trap Data" -> [w4579 _ w4613 w4652]
              tunnel: [w4579 w4594 w4613 w4652] -> w4483
              tunnel: w4482 -> [w4575 w4595 w4611 w4650]
              tunnel: w4481 -> [w4574 _ _ _]
              tunnel: [w4565 w4594 w4610 w4640] -> w4470
              tunnel: "Save Trap Pos. Data" -> [w4565 _ w4610 w4640]
              tunnel: w4473 -> [w4564 _ w4609 w4639]
              frame 1, Default {
                # "timeseries"
                n2845 = case shown="True" "Profile" {
                  tunnel: [w4588 w4592] -> w4569
                  tunnel: [w4588 w4591] -> w4568
                  tunnel: [w4588 w4590] -> w4567
                  tunnel: [w4588 w4589] -> w4566
                  frame False {
                    w4588 = 0.0 ("f")
                  }
                  frame True {
                    n2846 = local read "Current Position"() -> (w4593:cluster{dbl, dbl, dbl})
                    n2847 = local read "Y change (mm)"() -> (w4589:dbl)
                    n2848 = Unbundle(w4593) -> (w4592:dbl, w4591:dbl, w4590:dbl)
                  }
                }
                n2849 = local read "Save ave N"() -> (w4587:dbl)
                n2850 = Multiply(x=w4587, y=w4580) -> (x*y=w4586:dbl)
                n2851 = To Double Precision Float(number=w4564) -> (double precision float=w4578:dbl)
                n2852 = Build Array(w4575, w4580, w4586, w4585, w4584, 0.0 ("f")) -> (w4583:dbl[])
                n2853 = Build Array(w4578, w4569, w4568, w4567, w4566) -> (w4576:dbl[])
                n2854 = Select(t=u32 4000000000, s=w4574, f="N sets to save") -> (s? t:f=w4572:u32)
                n2855 = Build Array (concatenate)(w4583, w4582, w4576) -> (w4581:dbl[])
              }
              frame 2 {
                w4597 = 0.0 ("f")
                w4594 = FALSE ("Save APD Data\nwith Trap Data")
                # "calibration"
                n2856 = Boolean To (0,1)(Boolean=w4594) -> (0, 1=w4599:i16)
                n2857 = To Double Precision Float(number=w4599) -> (double precision float=w4598:dbl)
                n2858 = Build Array(w4598, w4597, w4597, w4597, w4597) -> (w4596:dbl[])
                n2859 = Build Array(w4595, w4600, w4600, w4607, w4606, 1.0 ("t")) -> (w4604:dbl[])
                n2860 = Build Array (concatenate)(w4604, w4603, w4596) -> (w4602:dbl[])
                "Calibrating Trap..." <- TRUE ("Calibrating...")
              }
              frame 4 {
                w4614 = 0.0 ("f")
                # "scan dir (x/y = 0/1)"
                # "cycles/step"
                # "n scans (f/b)"
                # "steps"
                # "freq. range"
                # "AOD raster scan"
                n2861 = local read "Number of F/B Scans (AOD)"() -> (w4621:u16)
                n2862 = local read "Cycles/step (AOD)"() -> (w4623:u64)
                n2863 = local read "Scan Range (MHz)"() -> (w4626:dbl)
                n2864 = local read "Scan steps (AOD)"() -> (w4625:u64)
                n2865 = local read "Scan BD"() -> (w4633:bool)
                n2866 = local read "Save ave N"() -> (w4638:dbl)
                n2867 = Boolean To (0,1)(Boolean=w4633) -> (0, 1=w4632:i16)
                n2868 = To Double Precision Float(number=w4621) -> (double precision float=w4620:dbl)
                n2869 = To Double Precision Float(number=w4625) -> (double precision float=w4624:dbl)
                n2870 = To Double Precision Float(number=w4623) -> (double precision float=w4622:dbl)
                n2871 = To Double Precision Float(number=w4632) -> (double precision float=w4631:dbl)
                n2872 = Multiply(x=w4638, y=w4616) -> (x*y=w4637:dbl)
                n2873 = To Double Precision Float(number=w4609) -> (double precision float=w4615:dbl)
                n2874 = Build Array(w4615, w4614, w4614, w4614, w4614) -> (w4612:dbl[])
                n2875 = local read "N sets should be saved"() -> (w4618:dbl)
                n2876 = Build Array(w4631, w4626, w4624, w4622, w4620) -> (w4628:dbl[])
                n2877 = Build Array(w4611, w4616, w4637, w4636, w4635, 2.0 ("t")) -> (w4630:dbl[])
                n2878 = Round Toward +Infinity(x=w4618) -> (ceil(x): smallest int >= x=w4619:dbl)
                n2879 = Build Array (concatenate)(w4630, w4629, w4612, w4628) -> (w4627:dbl[])
                n2880 = To Unsigned Long Integer(number=w4619) -> (unsigned 32bit integer=w4617:u32)
              }
              frame 8 {
                w4647 = 0.0 ("f")
                # "MCL raster scan"
                n2881 = local read "Number of scans (MCL)"() -> (w4642:u64)
                n2882 = local read "Scan lines (y)"() -> (w4641:u64)
                n2883 = local read "2D or 1D Scan"() -> (w4644:bool)
                n2884 = local read "Scan Range (V)\n(of steps)"() -> (w4663:dbl)
                n2885 = local read "Fast Scan Dir"() -> (w4670:bool)
                n2886 = local read "Cycles/step (MCL)"() -> (w4660:u64)
                n2887 = local read "Scan steps (MCL)"() -> (w4662:u64)
                n2888 = Select(t=w4641, s=w4644, f=w4642) -> (s? t:f=w4643:u64)
                n2889 = Boolean To (0,1)(Boolean=w4644) -> (0, 1=w4646:i16)
                n2890 = local read "Save ave N"() -> (w4675:dbl)
                n2891 = local read "Initial X"() -> (w4649:dbl)
                n2892 = local read "Initial Y"() -> (w4648:dbl)
                n2893 = To Double Precision Float(number=w4646) -> (double precision float=w4645:dbl)
                n2894 = Boolean To (0,1)(Boolean=w4670) -> (0, 1=w4669:i16)
                n2895 = To Double Precision Float(number=w4643) -> (double precision float=w4658:dbl)
                n2896 = To Double Precision Float(number=w4662) -> (double precision float=w4661:dbl)
                n2897 = To Double Precision Float(number=w4660) -> (double precision float=w4659:dbl)
                n2898 = To Double Precision Float(number=w4669) -> (double precision float=w4668:dbl)
                n2899 = Multiply(x=w4675, y=w4654) -> (x*y=w4674:dbl)
                n2900 = To Double Precision Float(number=w4639) -> (double precision float=w4653:dbl)
                n2901 = local read "N sets should be saved (MCL)"() -> (w4656:dbl)
                n2902 = Build Array(w4653, w4645, w4647, w4647, w4647) -> (w4651:dbl[])
                n2903 = Build Array(w4668, w4663, w4661, w4659, w4658, w4649, w4648) -> (w4665:dbl[])
                n2904 = Build Array(w4650, w4654, w4674, w4673, w4672, 3.0 ("t")) -> (w4667:dbl[])
                n2905 = Round Toward +Infinity(x=w4656) -> (ceil(x): smallest int >= x=w4657:dbl)
                n2906 = Build Array (concatenate)(w4667, w4666, w4651, w4665) -> (w4664:dbl[])
                n2907 = To Unsigned Long Integer(number=w4657) -> (unsigned 32bit integer=w4655:u32)
              }
            }
            n2908 = local read "Index"() -> (w4513:dbl)
            n2909 = call "Create new save file.vi"("Insert"="", "Ext"=".dat", "Index In"=w4513) -> ("Path Out"=w4472:path, "Index Out"=w4485:dbl)
            n2910 = local write "Save file name"(w4472) -> ()
            n2911 = local write "Index"(w4485) -> ()
            n2912 = local write "Save index"(w4485) -> ()
            n2913 = Array Size(array=w4496) -> (size(s)=w4497:i32)
            n2914 = Open/Create/Replace File(file path (use dialog)=w4472, operation (0:open)=T27."create", access (0:read/write)=enum16{"read/write", "read-only", "write-only"}."write-only") -> (refnum out=w4510:refnum<file>)  [unwired: 1 in, 4 out]
            n2915 = local write "Saving..."(TRUE ("Saving...")) -> ()
            n2916 = To Double Precision Float(number=w4497) -> (double precision float=w4495:dbl)
            n2917 = String Length(string="Comment (data description)") -> (length=w4493:i32)
            n2918 = To Double Precision Float(number=w4493) -> (double precision float=w4492:dbl)
            n2919 = Deny Access(7:w4510) -> (3:w4509:refnum<file>)  [unwired: 1 in, 2 out]
            n2920 = Build Array (concatenate)(w4495, w4496, w4492) -> (w4494:dbl[])
            n2921 = case "If fluorescence data to be saved" shown="True" w4483 {
              tunnel: w4472 -> [_ w4563]
              tunnel: [refnum<k0> refnum w4543] -> w4484
              frame False {
              }
              frame True {
                w4542 = 0.0
                n2922 = local read "APD Integration Time (s)"() -> (w4548:dbl)
                n2923 = local read "N APD Samp/step"() -> (w4541:dbl)
                n2924 = local read "Number of APDs"() -> (w4540:u8)
                n2925 = Path To String(path=w4563) -> (string=w4562:string)
                n2926 = String Length(string=w4562) -> (length=w4561:i32)
                n2927 = Subtract(x=w4561, y=4) -> (x-y=w4559:i32)
                n2928 = String Subset(string=w4562, length (rest)=w4559) -> (substring=w4558:string)  [unwired: 1 out]
                n2929 = Build Array(w4548, w4541, w4540, w4542, w4542, w4542, w4542, w4542) -> (w4545:dbl[])
                n2930 = Concatenate Strings(w4558, "_fl.dat" ("string")) -> (w4556:string)